vi "save_MPS_spectroscopy_hdf.vi"(0 "file path":path, 1 "Device Name":tag="DAQ2", 2 "Phase Rx over time":dbl[][](array[numeric]), 3 "Mag Rx over time":dbl[][](array[numeric]), 5 "TxRx_Params":T2={"sample rate"=1000000.0, "Tx freq"=23809.52380952381, "Tx amp"=1.5, "Tx cycles\nSpectroscopy"=500.0, "Bias amp"=2.0, "Bias freq"=11.904761904761905, "Receive range"=5.0, "Bias Periods\nMagnetometry"=5.0, "Tx Freq Division Factor"=42.0, "Drive Periods per Bias"=2000.0, "TX harmonics"=[52631.57894736842, 78947.36842105263, 105263.15789473684, 131578.94736842104, 157894.73684210525, 184210.52631578947, 210526.31578947368, 236842.1052631579]} {"TX harmonics" format="%#_6p"}, 7 "Rx_f0-f8 Units":string, 9 "Time Domain Cluster":T3={"Drive IMon"=array[500000 elements], "Rx Time Domain"=array[500000 elements], "Rx Empty Bore"=array[500000 elements], "BMon"=array[500000 elements], "Bias IMon"=array[500000 elements], "TF-Corr-MagOverTime"=[], "Interpolated Rx TF-Mag"=[], "Interpolated Rx TF-Phase"=[]}, 11 "Sample MetaData Cluster":T6={"Sample Volume (uL)"=5.0, "Sample Mass (ug)"=5.0, "Sample Conc(mg/mL)"=5.0, "Sample Temperature (C)"=5.0, "Batch Num"=5.0, "Batch Name"="", "Solute"="", "Solvent"="", "Sample Description"=""}, 12 "Study and Experiment Description":T5={"Study Number"=5, "Study Name"="", "UUID"="", "GUI Open Time"="", "Notes"=""}, 13 "Sample In Out Cluster":T1, 14 "Scanner Description":T4={"Scanner Name"="", "Hardware description"="", "Preamplifier Used"="", "Preamp Gain"=5.0, "Drive Amplifier"="", "Bias Amplifier"="", "Drive Current Monitor"="", "Bias Current Monitor"=""}, 15 "Points from home to max":i32) -> ()   [LabVIEW 2021]
uses:
  <vilib>/UPVI/lvhdf5/file.llb/LVH5F Operation.ctl
  <vilib>/Utility/miscctls.llb/LVRectTypeDef.ctl
  <vilib>/UPVI/lvhdf5/group.llb/H5G_obj_t.ctl
  <vilib>/UPVI/lvhdf5/dataset.llb/LVH5D Operation.ctl
  <vilib>/UPVI/lvhdf5/attribute.llb/LVH5A Operation.ctl
  <vilib>/UPVI/lvhdf5/identifier.llb/Not an HDF5 Refnum Constant.vi
  <vilib>/UPVI/lvhdf5/attribute.llb/Write Multiple Attributes.vi
  MPS_global_variables.vi
  <vilib>/UPVI/lvhdf5/utility.llb/Select HDF5 Dialog.vi
  <vilib>/UPVI/lvhdf5/utility.llb/Select HDF5 Dialog (Object Only).vi
  <vilib>/UPVI/lvhdf5/dataset.llb/Simple H5Dwrite (Variant).vi
  <vilib>/UPVI/lvhdf5/common.llb/To HDF5 Ref.vi
  <vilib>/UPVI/lvhdf5/dataset.llb/H5Dclose.vi
  <vilib>/UPVI/lvhdf5/attribute.llb/LVH5 Write Attributes.xnode
  <vilib>/UPVI/lvhdf5/library.llb/HDF5 Ref.ctl
  <vilib>/UPVI/lvhdf5/dataset.llb/Simple H5Dwrite.xnode
  <vilib>/UPVI/lvhdf5/dataset.llb/Write Dataset with Attributes.xnode
  <vilib>/UPVI/lvhdf5/attribute.llb/Cluster to Attribute Array.xnode
  <vilib>/Utility/error.llb/Error Cluster From Error Code.vi
  <vilib>/UPVI/lvhdf5/dataset.llb/OpenCreateReplace Dataset by Element Type.vi
  <vilib>/UPVI/lvhdf5/dataspace.llb/H5Sselect_hyperslab.vi
  <vilib>/UPVI/lvhdf5/dataset.llb/H5Dwrite (Variant).vi
  <vilib>/UPVI/lvhdf5/dataset.llb/H5Dget_space.vi
  <vilib>/UPVI/lvhdf5/attribute.llb/private/LVH5AwriteWDTAttrs.vi
  <vilib>/UPVI/lvhdf5/dataspace.llb/H5Sclose.vi
  <vilib>/UPVI/lvhdf5/utility.llb/Select HDF5 Dialog (File and Object).vi
  <resource>/objmgr/daqmx.rc
  <vilib>/UPVI/lvhdf5/library.llb/HDF5 Ref.lvclass
  <vilib>/Utility/Data Type/Get Type Information.vi
  <vilib>/Utility/Data Type/NI_Data Type.lvlib
  <vilib>/Utility/Data Type/Get Cluster Information.vi
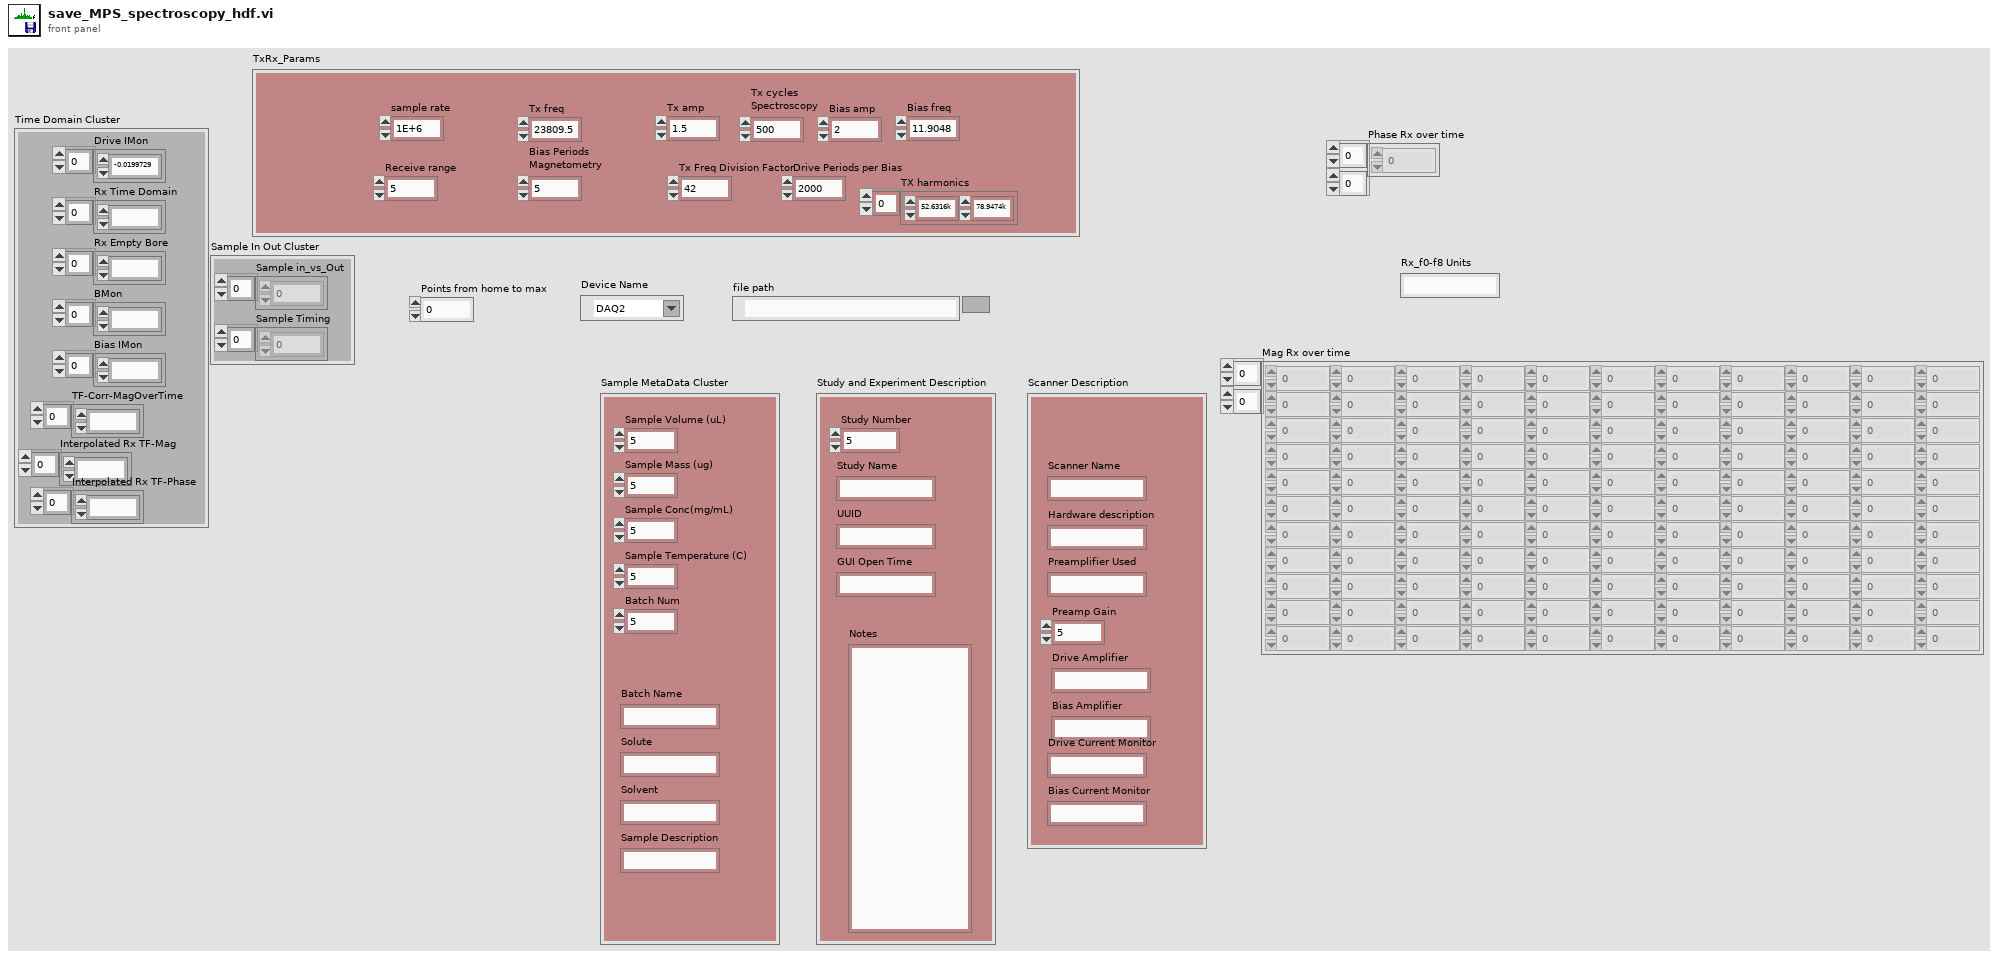
[diagram p1: front panel]
types:
  T1 = cluster{"Sample in_vs_Out":dbl[], "Sample Timing":dbl[]}
  T2 = cluster{"sample rate":dbl, "Tx freq":dbl, "Tx amp":dbl, "Tx cycles\nSpectroscopy":dbl, "Bias amp":dbl, "Bias freq":dbl, "Receive range":dbl, "Bias Periods\nMagnetometry":dbl, "Tx Freq Division Factor":dbl, "Drive Periods per Bias":dbl, "TX harmonics":dbl[]}
  T3 = cluster{"Drive IMon":dbl[], "Rx Time Domain":dbl[], "Rx Empty Bore":dbl[], "BMon":dbl[], "Bias IMon":dbl[], "TF-Corr-MagOverTime":dbl[], "Interpolated Rx TF-Mag":dbl[], "Interpolated Rx TF-Phase":dbl[]}
  T4 = cluster{"Scanner Name":string, "Hardware description":string, "Preamplifier Used":string, "Preamp Gain":dbl, "Drive Amplifier":string, "Bias Amplifier":string, "Drive Current Monitor":string, "Bias Current Monitor":string}
  T5 = cluster{"Study Number":i64, "Study Name":string, "UUID":string, "GUI Open Time":string, "Notes":string}
  T6 = cluster{"Sample Volume (uL)":dbl, "Sample Mass (ug)":dbl, "Sample Conc(mg/mL)":dbl, "Sample Temperature (C)":dbl, "Batch Num":dbl, "Batch Name":string, "Solute":string, "Solvent":string, "Sample Description":string}
  T7 = typedef "LVH5F Operation.ctl" = enum16{"open", "open or create", "create or replace", "create or replace (with confirmation)", "create", "open (read only)"}
  T8 = typedef "HDF5 Ref.ctl" = refnum<class "HDF5 Ref.lvclass">
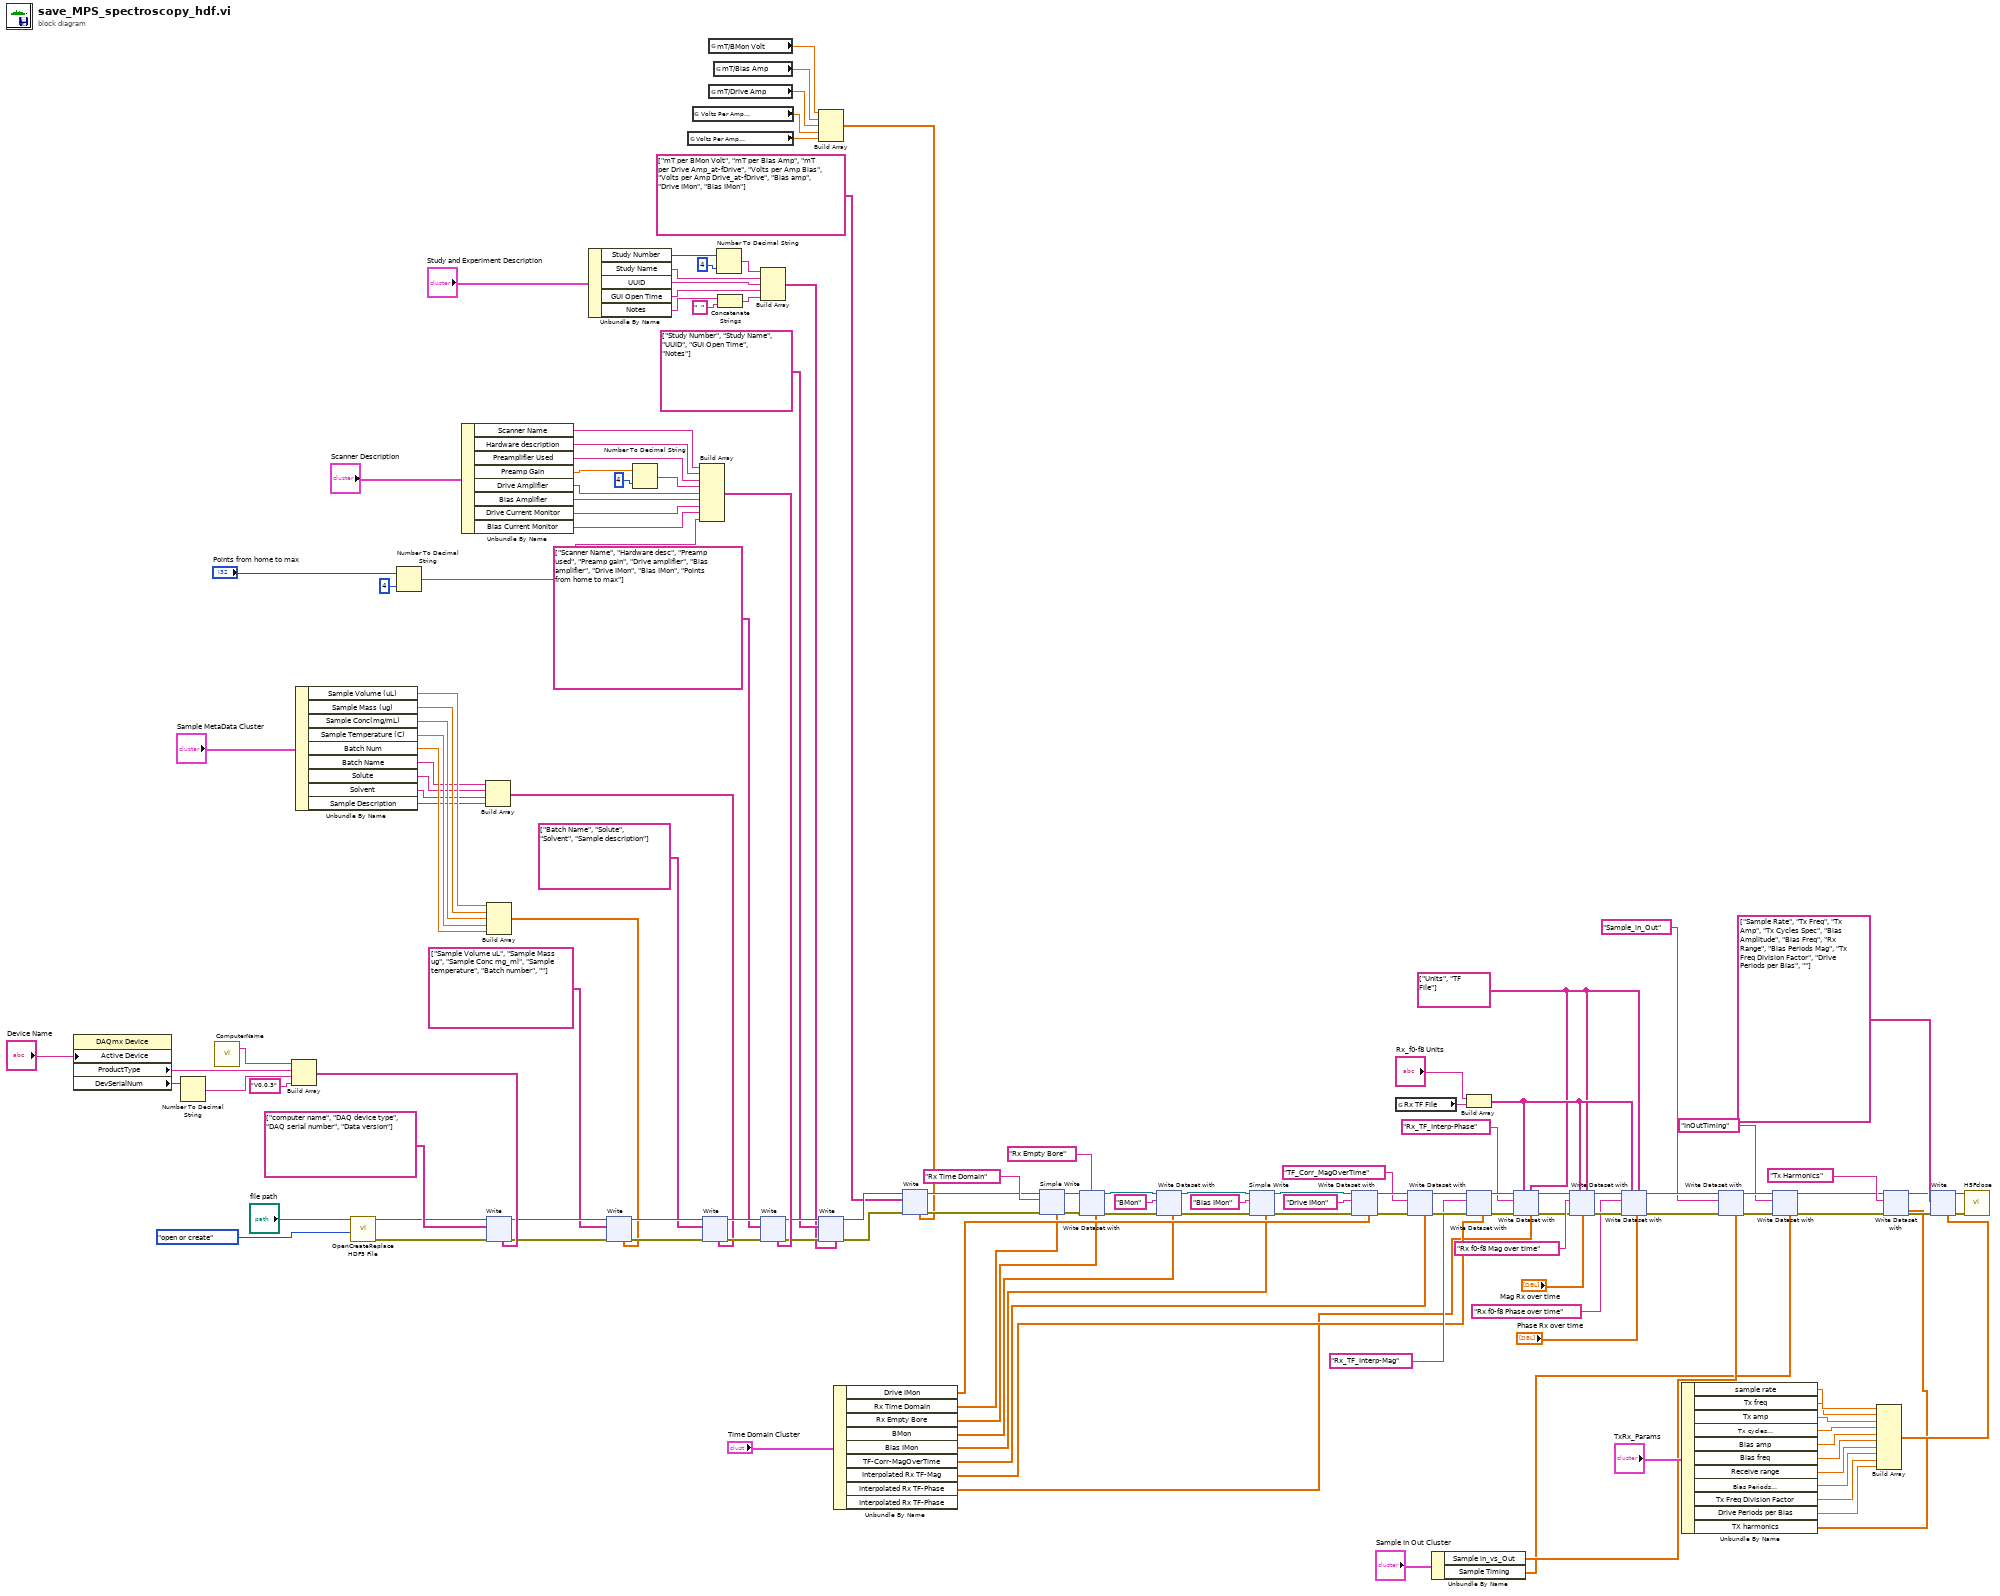
[diagram p0: block diagram]
diagram:
  w24 = string[] ["Units", "TF File"] ("Attribute Name(s)")
  n1 = property class="DAQmx Device"("Active Device"="Device Name") -> ("ProductType"=w139:string, "DevSerialNum"=w141:u32)  [unwired: 2 in, 2 out]
  n2 = Number To Decimal String(number=w141) -> (decimal integer string=w140:string)  [unwired: 1 in]
  n3 = call "ComputerName.vi"() -> ("String/Binary data"=w138:string)  [unwired: 4 in, 1 out]
  n4 = Build Array(w138, w139, w140, "V0.0.3" ("element")) -> (w137:string[])
  n5 = Unbundle By Name("Sample MetaData Cluster") -> ("Sample Volume (uL)"=w112:dbl, "Sample Mass (ug)"=w110:dbl, "Sample Conc(mg/mL)"=w109:dbl, "Sample Temperature (C)"=w108:dbl, "Batch Num"=w107:dbl, "Batch Name"=w106:string, "Solute"=w105:string, "Solvent"=w104:string, "Sample Description"=w103:string)
  n6 = call <vilib>:"OpenCreateReplace HDF5 File.vi"("function (open or create)"=LVH5F_Operation."open or create", "path"="file path") -> ("error out"=w132:errorcluster, "HDF5 Ref out"=w133:T8)  [unwired: 6 in]
  n7 = Number To Decimal String(number="Points from home to max", width (-)=i16 4) -> (decimal integer string=w10:string)
  n8 = Unbundle By Name("Scanner Description") -> ("Scanner Name"=w100:string, "Hardware description"=w99:string, "Preamplifier Used"=w98:string, "Preamp Gain"=w102:dbl, "Drive Amplifier"=w96:string, "Bias Amplifier"=w95:string, "Drive Current Monitor"=w94:string, "Bias Current Monitor"=w93:string)
  n9 = Build Array(w106, w105, w104, w103) -> (w84:string[])
  n10 = Build Array(w112, w110, w109, w108, w107) -> (w85:dbl[])
  n11 = xnode "Write"("HDF5 Ref"=w133, "error in (no error)"=w132, "Name(s)"=string[] ["computer name", "DAQ device type", "DAQ serial number", "Data version"], "Value(s)"=w137) -> ("HDF5 Ref out"=w131:T8, "error out"=w130:errorcluster)  [unwired: 1 in]
  n12 = Unbundle By Name("Study and Experiment Description") -> ("Study Number"=w91:i64, "Study Name"=w88:string, "UUID"=w87:string, "GUI Open Time"=w86:string, "Notes"=w39:string)
  n13 = xnode "Write"("HDF5 Ref"=w131, "error in (no error)"=w130, "Name(s)"=string[] ["Sample Volume uL", "Sample Mass ug", "Sample Conc mg_ml", "Sample temperature", "Batch number", ""], "Value(s)"=w85) -> ("HDF5 Ref out"=w119:T8, "error out"=w117:errorcluster)  [unwired: 1 in]
  n14 = Number To Decimal String(number=w102, width (-)=i16 4) -> (decimal integer string=w97:string)
  n15 = global read "MPS_global_variables.vi" "Volts Per Amp\nDrive"() -> (w15:dbl)
  n16 = global read "MPS_global_variables.vi" "Volts Per Amp\nBias"() -> (w16:dbl)
  n17 = Build Array(w100, w99, w98, w97, w96, w95, w94, w93, w10) -> (w83:string[])
  n18 = xnode "Write"("HDF5 Ref"=w119, "error in (no error)"=w117, "Name(s)"=string[] ["Batch Name", "Solute", "Solvent", "Sample description"], "Value(s)"=w84) -> ("HDF5 Ref out"=w118:T8, "error out"=w116:errorcluster)  [unwired: 1 in]
  n19 = global read "MPS_global_variables.vi" "mT/BMon Volt"() -> (w19:dbl)
  n20 = global read "MPS_global_variables.vi" "mT/Drive Amp"() -> (w17:dbl)
  n21 = global read "MPS_global_variables.vi" "mT/Bias Amp"() -> (w18:dbl)
  n22 = Number To Decimal String(number=w91, width (-)=i16 4) -> (decimal integer string=w89:string)
  n23 = Concatenate Strings(w39, "  " ("string")) -> (w38:string)
  n24 = Build Array(w89, w88, w87, w86, w38) -> (w79:string[])
  n25 = xnode "Write"("HDF5 Ref"=w118, "error in (no error)"=w116, "Name(s)"=string[] ["Scanner Name", "Hardware desc", "Preamp used", "Preamp gain", "Drive amplifier", "Bias amplifier", "Drive IMon", "Bias IMon", "Points from home to max"], "Value(s)"=w83) -> ("HDF5 Ref out"=w82:T8, "error out"=w81:errorcluster)  [unwired: 1 in]
  n26 = Build Array(w19, w18, w17, w16, w15) -> (w13:dbl[])
  n27 = xnode "Write"("HDF5 Ref"=w82, "error in (no error)"=w81, "Name(s)"=string[] ["Study Number", "Study Name", "UUID", "GUI Open Time", "Notes"], "Value(s)"=w79) -> ("HDF5 Ref out"=w23:T8, "error out"=w21:errorcluster)  [unwired: 1 in]
  n28 = Unbundle By Name("Time Domain Cluster") -> ("Drive IMon"=w77:dbl[], "Rx Time Domain"=w76:dbl[], "Rx Empty Bore"=w75:dbl[], "BMon"=w74:dbl[], "Bias IMon"=w73:dbl[], "TF-Corr-MagOverTime"=w40:dbl[], "Interpolated Rx TF-Mag"=w41:dbl[], "Interpolated Rx TF-Phase"=w27:dbl[])  [unwired: 1 out]
  n29 = xnode "Write"("HDF5 Ref"=w23, "error in (no error)"=w21, "Name(s)"=string[] ["mT per BMon Volt", "mT per Bias Amp", "mT per Drive Amp_at-fDrive", "Volts per Amp Bias", "Volts per Amp Drive_at-fDrive", "Bias amp", "Drive IMon", "Bias IMon"], "Value(s)"=w13) -> ("HDF5 Ref out"=w22:T8, "error out"=w20:errorcluster)  [unwired: 1 in]
  n30 = xnode "Simple Write"("Dataset Path"="Rx Time Domain", "error in (no error)"=w20, "HDF5 Path or Ref"=w22, "Data"=w76) -> ("HDF5 Ref out"=w143:T8, "error out"=w144:errorcluster)  [unwired: 4 in, 1 out]
  n31 = xnode "Write Dataset with"("Dataset Path"="Rx Empty Bore", "error in (no error)"=w144, "HDF5 Path or Ref"=w143, "Data"=w75) -> ("HDF5 Ref out"=w128:T8, "error out"=w127:errorcluster)  [unwired: 4 in, 1 out]
  n32 = xnode "Write Dataset with"("Dataset Path"="BMon", "error in (no error)"=w127, "HDF5 Path or Ref"=w128, "Data"=w74) -> ("HDF5 Ref out"=w125:T8, "error out"=w123:errorcluster)  [unwired: 4 in, 1 out]
  n33 = xnode "Simple Write"("Dataset Path"="Bias IMon", "error in (no error)"=w123, "HDF5 Path or Ref"=w125, "Data"=w73) -> ("HDF5 Ref out"=w124:T8, "error out"=w122:errorcluster)  [unwired: 4 in, 1 out]
  n34 = xnode "Write Dataset with"("Dataset Path"="Drive IMon", "error in (no error)"=w122, "HDF5 Path or Ref"=w124, "Data"=w77) -> ("HDF5 Ref out"=w44:T8, "error out"=w46:errorcluster)  [unwired: 4 in, 1 out]
  n35 = global read "MPS_global_variables.vi" "Rx TF File"() -> (w12:string)
  n36 = xnode "Write Dataset with"("Dataset Path"="TF_Corr_MagOverTime", "error in (no error)"=w46, "HDF5 Path or Ref"=w44, "Data"=w40) -> ("HDF5 Ref out"=w45:T8, "error out"=w47:errorcluster)  [unwired: 4 in, 1 out]
  n37 = Unbundle By Name("Sample In Out Cluster") -> ("Sample in_vs_Out"=w3:dbl[], "Sample Timing"=w2:dbl[])
  n38 = Build Array("Rx_f0-f8 Units", w12) -> (w25:string[])
  n39 = xnode "Write Dataset with"("Dataset Path"="Rx_TF_Interp-Mag", "error in (no error)"=w47, "HDF5 Path or Ref"=w45, "Data"=w41) -> ("HDF5 Ref out"=w32:T8, "error out"=w30:errorcluster)  [unwired: 4 in, 1 out]
  n40 = xnode "Write Dataset with"("Dataset Path"="Rx_TF_Interp-Phase", "error in (no error)"=w30, "HDF5 Path or Ref"=w32, "Attribute Name(s)"=w24, "Attribute Value(s)"=w25, "Data"=w27) -> ("HDF5 Ref out"=w31:T8, "error out"=w29:errorcluster)  [unwired: 2 in, 1 out]
  n41 = xnode "Write Dataset with"("Dataset Path"="Rx f0-f8 Mag over time", "error in (no error)"=w29, "HDF5 Path or Ref"=w31, "Attribute Name(s)"=w24, "Attribute Value(s)"=w25, "Data"="Mag Rx over time") -> ("HDF5 Ref out"=w55:T8, "error out"=w54:errorcluster)  [unwired: 2 in, 1 out]
  n42 = xnode "Write Dataset with"("Dataset Path"="Rx f0-f8 Phase over time", "error in (no error)"=w54, "HDF5 Path or Ref"=w55, "Attribute Name(s)"=w24, "Attribute Value(s)"=w25, "Data"="Phase Rx over time") -> ("HDF5 Ref out"=w51:T8, "error out"=w50:errorcluster)  [unwired: 2 in, 1 out]
  n43 = Unbundle By Name("TxRx_Params") -> ("sample rate"=w70:dbl, "Tx freq"=w69:dbl, "Tx amp"=w68:dbl, "Tx cycles\nSpectroscopy"=w67:dbl, "Bias amp"=w66:dbl, "Bias freq"=w65:dbl, "Receive range"=w64:dbl, "Bias Periods\nMagnetometry"=w63:dbl, "Tx Freq Division Factor"=w57:dbl, "Drive Periods per Bias"=w58:dbl, "TX harmonics"=w33:dbl[])
  n44 = xnode "Write Dataset with"("Dataset Path"="Sample_in_Out", "error in (no error)"=w50, "HDF5 Path or Ref"=w51, "Data"=w3) -> ("HDF5 Ref out"=w5:T8, "error out"=w8:errorcluster)  [unwired: 4 in, 1 out]
  n45 = xnode "Write Dataset with"("Dataset Path"="InOutTiming", "error in (no error)"=w8, "HDF5 Path or Ref"=w5, "Data"=w2) -> ("HDF5 Ref out"=w6:T8, "error out"=w7:errorcluster)  [unwired: 4 in, 1 out]
  n46 = Build Array(w70, w69, w68, w67, w66, w65, w64, w63, w57, w58) -> (w56:dbl[])
  n47 = xnode "Write Dataset with"("Dataset Path"="Tx Harmonics", "error in (no error)"=w7, "HDF5 Path or Ref"=w6, "Data"=w33) -> ("HDF5 Ref out"=w35:T8, "error out"=w36:errorcluster)  [unwired: 4 in, 1 out]
  n48 = xnode "Write"("HDF5 Ref"=w35, "error in (no error)"=w36, "Name(s)"=string[] ["Sample Rate", "Tx Freq", "Tx Amp", "Tx Cycles Spec", "Bias Amplitude", "Bias Freq", "Rx Range", "Bias Periods Mag", "Tx Freq Division Factor", "Drive Periods per Bias", ""], "Value(s)"=w56) -> ("HDF5 Ref out"=w72:T8, "error out"=w62:errorcluster)  [unwired: 1 in]
  n49 = call <vilib>:"H5Fclose.vi"("error in (no error)"=w62, "HDF5 Ref"=w72) -> ()  [unwired: 7 in, 1 out]
